vi "FlexMag - 23-03-2023.vi"() -> ()   [LabVIEW 2018] (continued)
  in  "Tp3 auto set speed":bool
  in  "Tp3 auto stop":bool
  in  "Tp3 auto start":bool
  in  "Tp4 auto normal speed":bool
  in  "Tp4 auto low speed":bool
  in  "Tp4 auto set speed":bool
  in  "Tp4 auto stop":bool
  in  "Tp4 auto start":bool
  in  "Tp1 Stop initial":bool
  in  "Tp1 Start initial":bool
  in  "Tp2 stop initial":bool
  in  "Tp2 start initial":bool
  in  "Tp3 stop initial":bool
  in  "Tp3 start initial":bool
  in  "Tp4 stop initial":bool
  in  "Tp4 start initial":bool
  out "Tp1_stop_cmnd":bool
  out "Tp2_stop_cmnd":bool
  out "Tp3_stop_cmnd":bool
  out "Tp4_stop_cmnd":bool
  out "tp1 com":bool
  out "tp2 com":bool
  out "tp3 com":bool
  out "tp4 com":bool
  in  "Adress set":bool
  out "after substring":string
  out "after substring 2":string
  out "after substring 3":string
  out "after substring 4":string
  out "tp3 readout":string
  out "tp2 readout":string
  out "tp1 readout":string
  out "tp4 readout":string
  in  "Baratron1 auto set zero":bool
  in  "pcgv1 auto set pressure":bool
  in  "pcgv1 auto close":bool
  in  "pcgv1 auto open":bool
  in  "pcgv1 auto set position":bool
  in  "Baratron2 auto set zero":bool
  in  "pcgv2 auto set pressure":bool
  in  "pcgv2 auto close":bool
  in  "pcgv2 auto set position":bool
  in  "pcgv2 auto open":bool
  in  "pcgv3 auto close":bool
  in  "pcgv3 auto set pressure":bool
  in  "pcgv3 auto set position":bool
  in  "Baratron3 set zero gui":bool
  in  "pcgv3 auto open":bool
  in  "Baratron4 auto set zero":bool
  in  "pcgv4 auto set pressure":bool
  in  "pcgv4 auto set position":bool
  in  "pcgv4 auto close":bool
  in  "pcgv4 auto open":bool
  out "pcgv1 setted pressure value torr":dbl
  out "pcgv2 setted pressure value torr":dbl
  out "pcgv3 setted pressure value torr":dbl
  out "pcgv4 setted pressure value torr":dbl
  in  "pcgv1 close gui 2":bool
  in  "pcgv1 open gui 2":bool
  in  "pcgv2 close gui 2":bool
  in  "pcgv2 open gui 2":bool
  in  "pcgv3 close gui 2":bool
  in  "pcgv3 open gui 2":bool
  in  "pcgv4 open gui 2":bool
  in  "pcgv4 close gui 2":bool
  in  "string":string
  in  "Learn":bool
  in  "Learn value":string
  out "Pressure_gui 2":dbl format="%.1f"
  out "Pressure_gui":dbl format="%.1f"
  out "Pressure":dbl format="%.1f"
  out "Pressure 2_gui 2":i32 format="%.1f"
  out "Pressure 2_gui":i32 format="%.1f"
  out "Pressure 2":i32 format="%.1f"
  out "Pressure ch3_gui2":i32 format="%.1f"
  out "Pressure ch3_gui":i32 format="%.1f"
  out "Pressure_ch3":i32
  out "Pressurech4_gui 2":i32 format="%.1f"
  out "Pressurech4_gui":i32 format="%.1f"
  out "Pressure 4":i32
  in  "Counter Data set":i16
  in  "Counter data set":bool
  out "Counter Read Data":i16
  out "CH1 CH BG":string
  out "CH2 CH BG":string
  out "CH4 CH BG":string
  out "CH3 CH BG":string
  out "CH1 CH CC":string
  out "CH1 CH PG":string
  out "ch4 pl pg torr":dbl format="%#_2e"
  out "ch4 pl pg mbar":dbl format="%#_2e"
  out "ch4 ch pg mbar":dbl format="%#_2e"
  out "ch4 ch pg torr":dbl format="%#_2e"
  out "ch4 cc torr":dbl format="%#_2e"
  out "ch4 cc mbar":dbl format="%#_2e"
  out "ch3 cc torr":dbl format="%#_2e"
  out "ch3 cc mbar":dbl format="%#_2e"
  out "ch3 ch pg torr":dbl format="%#_2e"
  out "ch3 ch pg mbar":dbl format="%#_2e"
  out "ch3 pl pg  torr":dbl format="%#_2e"
  out "ch3 pl pg mbar":dbl format="%#_2e"
  out "ch2 pl pg  torr":dbl format="%#_2e"
  out "ch2 pl pg mbar":dbl format="%#_2e"
  out "ch2 ch pg mbar":dbl format="%#_2e"
  out "ch2 ch pg torr":dbl format="%#_2e"
  out "ch2 cc torr":dbl format="%#_2e"
  out "ch2 cc mbar":dbl format="%#_2e"
  out "ch1 pl pg  torr":dbl format="%#_2e"
  out "ch1 pl pg mbar":dbl format="%#_2e"
  out "ch1 ch pg torr":dbl format="%#_2e"
  out "ch1 ch pg mbar":dbl format="%#_2e"
  out "ch1 cc torr":dbl format="%#_2e"
  out "ch1 cc mbar":dbl format="%#_2e"
  out "ch4 pl pg mbar gui 1":dbl format="%#_2e"
  out "ch3 pl pg mbar gui 1":dbl format="%#_2e"
  out "ch2 pl pg mbar gui 1":dbl format="%#_2e"
  out "ch1 pl pg mbar gui 1":dbl format="%#_2e"
  out "ch3 pl pg ai(V)":dbl
  out "ch3 ch pg ai(V)":dbl
  out "ch3 cc ai(V)":dbl
  out "ch2 pl pg ai(V)":dbl
  out "ch2 ch pg ai(V)":dbl
  out "ch2 cc ai(V)":dbl
  out "ch1 cc ai(V)":dbl
  out "ch1 ch pg ai(V)":dbl
  out "ch1 pl pg ai(V)":dbl
  out "ch4 pl pg ai(V)":dbl
  out "ch4 ch pg ai(V)":dbl
  out "ch4 cc ai(V)":dbl
  out "iteration for graph":i32
  out "hour s":string
  out "min s":string
  out "sec s":string
  out "hour":i32
  out "min":i32
  out "sec":i32
  out "time string":string
  out "CH1 PL PG":string
  out "CH2 CH CC":string
  out "CH2 CH PG":string
  out "CH2 PL PG":string
  out "CH4 CH CC":string
  out "CH4 CH PG":string
  out "CH4 PL PG":string
  out "CH3 CH CC":string
  out "CH3 CH PG":string
  out "CH3 PL PG":string
  in  "time  (sec)":u32
  in  "ch4 sd clear":bool
  in  "ch3 sd clear":bool
  in  "ch2 sd clear":bool
  in  "ch1 sd clear":bool
  in  "ch4 pd clear":bool
  in  "ch3 pd clear":bool
  in  "ch2 pd clear":bool
  in  "ch1 pd clear":bool
  out "ch1 pd continue":bool
  out "ch1 pd cancel":bool
  out "ch2 pd cancel":bool
  out "ch2 pd continue":bool
  out "ch3 pd cancel":bool
  out "ch3 pd continue":bool
  out "ch4 pd cancel":bool
  out "ch4 pd continue":bool
  out "ch1 sd cancel":bool
  out "ch1 sd continue":bool
  in  "ch1 shutdown alg":bool
  in  "ch2 shutdown alg":bool
  in  "ch4 shutdown alg":bool
  in  "ch3 shutdown alg":bool
  out "ch2 sd cancel":bool
  out "ch2 sd continue":bool
  out "ch3 sd cancel":bool
  out "ch3 sd continue":bool
  out "ch4 sd cancel":bool
  out "ch4 sd continue":bool
  in  "abort ch1":bool
  in  "abort ch2":bool
  in  "abort ch4":bool
  in  "abort ch3":bool
  in  "ch1 pumpdown alg":bool
  in  "ch2 pumpdown alg":bool
  in  "ch4 pumpdown alg":bool
  in  "ch3 pumpdown alg":bool
  in  "ch1 pumpdown error":bool
  in  "ch2 pumpdown error":bool
  in  "ch4 pumpdown error":bool
  in  "ch3 pumpdown error":bool
  in  "ch4 shutdown error":bool
  in  "ch3 shutdown error":bool
  in  "ch2 shutdown error":bool
  in  "ch1 shutdown error":bool
  out "ch1 vent?":bool
  out "ch2 vent?":bool
  out "ch3 vent?":bool
  out "ch4 vent?":bool
  out "ch1 atms close led":bool
  out "ch1 ch vbv close led":bool
  out "ch1 tp bv open led":bool
  out "ch1 pl vbv close led":bool
  out "ch1-ch2 trns gv close led 2":bool
  out "ch1 trns bp left close led":bool
  out "ch1 mp start led":bool
  out "ch1 pc gv open led":bool
  out "ch1 pl press under 0.05 T led":bool
  out "ch1 ch press under 0.5 T led":bool
  out "ch1 tp start led":bool
  out "ch1 trns bp left open led":bool
  out "ch1 ch press under 0.01 T led":bool
  out "ch1 cc open led":bool
  out "ch1 desired pressure led":bool
  out "ch1 pd completed led":bool
  out "ch1 sd completed led":bool
  out "ch1 sd PL-CH atm on led":bool
  out "ch1 sd PL atm on led":bool
  out "ch1 sd trns bp left close led":bool
  out "ch1 sd ch vbv open led":bool
  out "ch1 sd trns bp left open led":bool
  out "ch1 sd pcgv close led":bool
  out "ch1 sd atms close led":bool
  out "ch1 sd tp bv close led":bool
  out "ch1 sd pcgv open led":bool
  out "ch1 sd pl vbv open led":bool
  out "ch1 sd mp stop led":bool
  out "ch1 sd bg bv close led":bool
  out "ch1 sd tp stop led":bool
  out "ch1 sd cc close led":bool
  out "ch2 desired pressure led":bool
  out "ch2 cc open led":bool
  out "ch2 ch press under 0.01 T led":bool
  out "ch2 trns bp left open led":bool
  out "ch2 tp start led":bool
  out "ch2 ch press under 0.5 T led":bool
  out "ch2 pl press under 0.05 T led":bool
  out "ch1-ch2 trns gv close led":bool
  out "ch2 trns bp left close led":bool
  out "ch2 mp start led":bool
  out "ch2 pc gv open led":bool
  out "ch2 tp bv open led":bool
  out "ch2 pl vbv close led":bool
  out "ch2 ch vbv close led":bool
  out "ch2 atms close led":bool
  out "ch2 pd completed led":bool
  out "ch2 trns bp right close led":bool
  out "ch2 trns bp right open led":bool
  out "ch2-ch3 trns gv close led":bool
  out "ch2 sd completed led":bool
  out "ch2 sd PL-CH atm on led":bool
  out "ch2 sd PL atm on led":bool
  out "ch2 sd trns bp left close led":bool
  out "ch2 sd ch vbv open led":bool
  out "ch2 sd trns bp left open led":bool
  out "ch2 sd pcgv close led":bool
  out "ch2 sd atms close led":bool
  out "ch2 sd tp bv close led":bool
  out "ch2 sd pcgv open led":bool
  out "ch2 sd pl vbv open led":bool
  out "ch2 sd mp stop led":bool
  out "ch2 sd bg bv close led":bool
  out "ch2 sd tp stop led":bool
  out "ch2 sd cc close led":bool
  out "ch2 sd trns bp right close led":bool
  out "ch2 sd trns bp right open led":bool
  out "ch3 trns bp right open led":bool
  out "ch3 trns bp right close led":bool
  out "ch3 pd completed led":bool
  out "ch3 desired pressure led":bool
  out "ch3 cc open led":bool
  out "ch3 ch press under 0.01 T led":bool
  out "ch3 trns bp left open led":bool
  out "ch3 tp start led":bool
  out "ch3 ch press under 0.5 T led":bool
  out "ch3 pl press under 0.05 T led":bool
  out "ch3-ch2 trns gv close led":bool
  out "ch3 trns bp left close led":bool
  out "ch3 mp start led":bool
  out "ch3 pc gv open led":bool
  out "ch3 tp bv open led":bool
  out "ch3 pl vbv close led":bool
  out "ch3 ch vbv close led":bool
  out "ch3 atms close led":bool
  out "ch3-ch4 trns gv close led":bool
  out "ch4-ch3 trns gv close led":bool
  out "ch4 trns bp right open led":bool
  out "ch4 trns bp right close led":bool
  out "ch4 pd completed led":bool
  out "ch4 desired pressure led":bool
  out "ch4 cc open led":bool
  out "ch4 ch press under 0.01 T led":bool
  out "ch4 tp start led":bool
  out "ch4 ch press under 0.5 T led":bool
  out "ch4 pl press under 0.05 T led":bool
  out "ch4 mp start led":bool
  out "ch4 pc gv open led":bool
  out "ch4 tp bv open led":bool
  out "ch4 pl vbv close led":bool
  out "ch4 ch vbv close led":bool
  out "ch4 atms close led":bool
  out "ch3 sd trns bp right close led":bool
  out "ch3 sd trns bp right open led":bool
  out "ch3 sd completed led":bool
  out "ch3 sd PL-CH atm on led":bool
  out "ch3 sd PL atm on led":bool
  out "ch3 sd trns bp left close led":bool
  out "ch3 sd ch vbv open led":bool
  out "ch3 sd trns bp left open led":bool
  out "ch3 sd pcgv close led":bool
  out "ch3 sd atms close led":bool
  out "ch3 sd tp bv close led":bool
  out "ch3 sd pcgv open led":bool
  out "ch3 sd pl vbv open led":bool
  out "ch3 sd mp stop led":bool
  out "ch3 sd bg bv close led":bool
  out "ch3 sd tp stop led":bool
  out "ch3 sd cc close led":bool
  out "ch4 sd completed led":bool
  out "ch4 sd PL-CH atm on led":bool
  out "ch4 sd PL atm on led":bool
  out "ch4 sd trns bp right close led":bool
  out "ch4 sd ch vbv open led":bool
  out "ch4 sd trns bp right open led":bool
  out "ch4 sd pcgv close led":bool
  out "ch4 sd atms close led":bool
  out "ch4 sd tp bv close led":bool
  out "ch4 sd pcgv open led":bool
  out "ch4 sd pl vbv open led":bool
  out "ch4 sd mp stop led":bool
  out "ch4 sd bg bv close led":bool
  out "ch4 sd tp stop led":bool
  out "ch4 sd cc close led":bool
  in  "ch1 ar set zero auto":bool
  in  "ch1 ar set auto":bool
  in  "ch3 ar set auto":bool
  in  "ch2 ar set auto":bool
  in  "ch3 ar set zero auto":bool
  in  "ch2 ar set zero auto":bool
  in  "ch4 ar set zero auto":bool
  in  "ch4 ar set auto":bool
  in  "dewar error time(min)":dbl=10.0
  in  "error level":dbl=30.0
  in  "ln2 ch4 bottom drop":dbl=35.0
  in  "ln2 ch4 top aim":dbl=39.0
  in  "ln2 ch3 bottom drop":dbl=35.0
  in  "ln2 ch3 top aim":dbl=39.0
  in  "ln2 ch1 bottom drop":dbl=35.0
  in  "ln2 ch1 top aim":dbl=39.0
  in  "ln2 ch2 bottom drop":dbl=35.0
  in  "ln2 ch2 top aim":dbl=39.0
  in  "ln2 dropdown":dbl=32.0
  in  "GUI_inputs":enum32{"CH1", "CH2", "CH3", "CH4", "Others"}(tab)
  in  "ch1_mp_gui":bool
  in  "ch1_mp_fail":bool
  in  "ch1_pl_vbv_fail":bool
  in  "ch1_pl_vbv_gui":bool
  in  "ch1_pl_atm_fail":bool
  in  "ch1_pl_atm_gui":bool
  in  "ch1_pl_pg_fail":bool
  in  "ch1_pl_pg_gui":bool
  in  "ch1_tp_bv_fail":bool
  in  "ch1_tp_bv_gui":bool
  in  "ch1_ch_vbv_fail":bool
  in  "ch1_ch_vbv_gui":bool
  in  "ch1_tp_fail":bool
  in  "ch1_tp_gui":bool
  in  "ch1_pcgv_gui":bool
  in  "ch1_pcgv_half_gui":bool
  in  "ch1_pcgv_fail":bool
  in  "ch1_ch_pg_fail":bool
  in  "ch1_ch_pg_gui":bool
  in  "ch1_cc_fail":bool
  in  "ch1_cc_gui":bool
  in  "ch1_bg_fail":bool
  in  "ch1_bg_gui":bool
  in  "ch1_bg_bv_fail":bool
  in  "ch1_bg_bv_gui":bool
  in  "ch1_ch_atm_fail":bool
  in  "ch1_ch_atm_gui":bool
  in  "ch1_sov_fail":bool
  in  "ch1_sov_gui":bool
  in  "ch2_mp_fail":bool
  in  "ch2_mp_gui":bool
  in  "ch2_pl_vbv_fail":bool
  in  "ch2_pl_vbv_gui":bool
  in  "ch2_pl_atm_fail":bool
  in  "ch2_pl_atm_gui":bool
  in  "ch2_pl_pg_fail":bool
  in  "ch2_pl_pg_gui":bool
  in  "ch2_tp_bv_fail":bool
  in  "ch2_tp_bv_gui":bool
  in  "ch2_ch_vbv_fail":bool
  in  "ch2_ch_vbv_gui":bool
  in  "ch2_tp_fail":bool
  in  "ch2_tp_gui":bool
  in  "ch2_pcgv_gui":bool
  in  "ch2_pcgv_half_gui":bool
  in  "ch2_pcgv_fail":bool
  in  "ch2_ch_pg_fail":bool
  in  "ch2_ch_pg_gui":bool
  in  "ch2_cc_fail":bool
  in  "ch2_cc_gui":bool
  in  "ch2_bg_fail":bool
  in  "ch2_bg_gui":bool
  in  "ch2_bg_bv_fail":bool
  in  "ch2_bg_bv_gui":bool
  in  "ch2_ch_atm_fail":bool
  in  "ch2_ch_atm_gui":bool
  in  "ch2_sov_fail":bool
  in  "ch2_sov_gui":bool
  in  "ch3_mp_fail":bool
  in  "ch3_mp_gui":bool
  in  "ch3_pl_vbv_fail":bool
  in  "ch3_pl_vbv_gui":bool
  in  "ch3_pl_atm_fail":bool
  in  "ch3_pl_atm_gui":bool
  in  "ch3_pl_pg_fail":bool
  in  "ch3_pl_pg_gui":bool
  in  "ch3_tp_bv_fail":bool
  in  "ch3_tp_bv_gui":bool
  in  "ch3_ch_vbv_fail":bool
  in  "ch3_ch_vbv_gui":bool
  in  "ch3_tp_fail":bool
  in  "ch3_tp_gui":bool
  in  "ch3_pcgv_half_gui":bool
  in  "ch3_pcgv_gui":bool
  in  "ch3_pcgv_fail":bool
  in  "ch3_ch_pg_fail":bool
  in  "ch3_ch_pg_gui":bool
  in  "ch3_cc_fail":bool
  in  "ch3_cc_gui":bool
  in  "ch3_bg_fail":bool
  in  "ch3_bg_gui":bool
  in  "ch3_bg_bv_fail":bool
  in  "ch3_bg_bv_gui":bool
  in  "ch3_ch_atm_fail":bool
  in  "ch3_ch_atm_gui":bool
  in  "ch3_sov_fail":bool
  in  "ch3_sov_gui":bool
  in  "ch4_mp_fail":bool
  in  "ch4_mp_gui":bool
  in  "ch4_pl_vbv_fail":bool
  in  "ch4_pl_vbv_gui":bool
  in  "ch4_pl_atm_fail":bool
  in  "ch4_pl_atm_gui":bool
  in  "ch4_pl_pg_fail":bool
  in  "ch4_pl_pg_gui":bool
  in  "ch4_tp_bv_fail":bool
  in  "ch4_tp_bv_gui":bool
  in  "ch4_ch_vbv_fail":bool
  in  "ch4_ch_vbv_gui":bool
  in  "ch4_tp_fail":bool
  in  "ch4_tp_gui":bool
  in  "ch4_pcgv_gui":bool
  in  "ch4_pcgv_half_gui":bool
  in  "ch4_pcgv_fail":bool
  in  "ch4_ch_pg_fail":bool
  in  "ch4_ch_pg_gui":bool
  in  "ch4_cc_fail":bool
  in  "ch4_cc_gui":bool
  in  "ch4_bg_fail":bool
  in  "ch4_bg_gui":bool
  in  "ch4_bg_bv_fail":bool
  in  "ch4_bg_bv_gui":bool
  in  "ch4_ch_atm_fail":bool
  in  "ch4_ch_atm_gui":bool
  in  "ch4_sov_fail":bool
  in  "ch4_sov_gui":bool
  in  "ch3_4_trns_gv_fail":bool
  in  "ch3_4_trns_gv_gui":bool
  in  "ch2_3_trns_gv_fail":bool
  in  "ch2_3_trns_gv_gui":bool
  in  "ch1_2_trns_gv_fail":bool
  in  "ch1_2_trns_gv_gui":bool
  in  "ch4_gv_bp_right_fail":bool
  in  "ch4_gv_bp_right_gui":bool
  in  "ch3_gv_bp_right_fail":bool
  in  "ch3_gv_bp_right_gui":bool
  in  "ch2_gv_bp_right_fail":bool
  in  "ch2_gv_bp_right_gui":bool
  in  "ch3_gv_bp_left_fail":bool
  in  "ch3_gv_bp_left_gui":bool
  in  "ch2_gv_bp_left_fail":bool
  in  "ch2_gv_bp_left_gui":bool
  in  "ch1_gv_bp_left_fail":bool
  in  "ch1_gv_bp_left_gui":bool
  in  "casette_ch1_gui":bool
  in  "casette_ch3_gui":bool
  in  "casette_ch2_gui":bool
  in  "casette_ch4_gui":bool
  in  "24-bit pixmap tab":enum32{"Page 1", "Page 2", "Page 3", "Page 4"}(tab)
  out "main screen jpeg":u32[][](array[numeric]) format="%x"
  out "pl pg fail jpeg":u32[][](array[numeric]) format="%x"
  out "pl pg on jpeg":u32[][](array[numeric]) format="%x"
  out "pc gv half jpeg":u32[][](array[numeric]) format="%x"
  out "cc fail jpeg":u32[][](array[numeric]) format="%x"
  out "cc on jpeg":u32[][](array[numeric]) format="%x"
  out "gv bp left fail jpeg":u32[][](array[numeric]) format="%x"
  out "gv bp left on jpeg":u32[][](array[numeric]) format="%x"
  out "tp bv fail jpeg":u32[][](array[numeric]) format="%x"
  out "tp bv on jpeg":u32[][](array[numeric]) format="%x"
  out "pc gv fail jpeg":u32[][](array[numeric]) format="%x"
  out "pc gv on jpeg":u32[][](array[numeric]) format="%x"
  out "bg fail jpeg":u32[][](array[numeric]) format="%x"
  out "bg on jpeg":u32[][](array[numeric]) format="%x"
  out "gv bp right fail jpeg":u32[][](array[numeric]) format="%x"
  out "gv bp right on jpeg":u32[][](array[numeric]) format="%x"
  out "ch pg on jpeg":u32[][](array[numeric]) format="%x"
  out "ch pg fail jpeg":u32[][](array[numeric]) format="%x"
  out "pl atm on jpeg":u32[][](array[numeric]) format="%x"
  out "pl atm fail jpeg":u32[][](array[numeric]) format="%x"
  out "ch atm on jpeg":u32[][](array[numeric]) format="%x"
  out "ch atm fail jpeg":u32[][](array[numeric]) format="%x"
  out "tp start jpeg":u32[][](array[numeric]) format="%x"
  out "tp fail jpeg":u32[][](array[numeric]) format="%x"
  out "pl vbv fail jpeg":u32[][](array[numeric]) format="%x"
  out "pl vbv on jpeg":u32[][](array[numeric]) format="%x"
  out "bg bv on jpeg":u32[][](array[numeric]) format="%x"
  out "bg bv fail jpeg":u32[][](array[numeric]) format="%x"
  out "tp vbv on jpeg":u32[][](array[numeric]) format="%x"
  out "tp vbv fail jpeg":u32[][](array[numeric]) format="%x"
  out "mp on jpeg":u32[][](array[numeric]) format="%x"
  out "mp fail jpeg":u32[][](array[numeric]) format="%x"
  out "trns gv fail jpeg":u32[][](array[numeric]) format="%x"
  out "trns gv on jpeg":u32[][](array[numeric]) format="%x"
  out "ch1 top main jpeg":u32[][](array[numeric]) format="%x"
  out "ch1 front main jpeg":u32[][](array[numeric]) format="%x"
  out "ch2 front main jpeg":u32[][](array[numeric]) format="%x"
  out "ch2 top main jpeg":u32[][](array[numeric]) format="%x"
  out "ch3 front main jpeg":u32[][](array[numeric]) format="%x"
  out "ch3 top main jpeg":u32[][](array[numeric]) format="%x"
  out "ch4 front main jpeg":u32[][](array[numeric]) format="%x"
  out "ch4 top main jpeg":u32[][](array[numeric]) format="%x"
  out "sov fail jpeg":u32[][](array[numeric]) format="%x"
  out "sov on jpeg":u32[][](array[numeric]) format="%x"
  out "trns gv top right fail jpeg":u32[][](array[numeric]) format="%x"
  out "trns gv top right on  jpeg":u32[][](array[numeric]) format="%x"
  out "trns gv front left on jpeg":u32[][](array[numeric]) format="%x"
  out "trns gv front left fail jpeg":u32[][](array[numeric]) format="%x"
  out "trns gv front right on jpeg":u32[][](array[numeric]) format="%x"
  out "trns gv front right fail jpeg":u32[][](array[numeric]) format="%x"
  out "trns gv top left fail jpeg":u32[][](array[numeric]) format="%x"
  out "trns gv top left on jpeg":u32[][](array[numeric]) format="%x"
  out "casette jpeg":u32[][](array[numeric]) format="%x"
  out "trns sensors led":bool
  in  "deactivate all trns sensors":bool
  in  "Cst_Speed_Low":dbl=500.0
  out "trns V?":bool
  out "trns 2-3 led 1":bool
  out "trns 2-3 led 4":bool
  out "trns 2-3 led 6":bool
  out "trns 2-3 led 8":bool
  out "trns 2-3 led 2":bool
  out "trns 2-3 led 3":bool
  out "trns 2-3 led 5":bool
  out "trns 2-3 led 7":bool
  out "trns 2-3 led 9":bool
  out "trns 2-3 led 10":bool
  out "trns 2-3 led 11":bool
  out "trns 2-3 led 12":bool
  out "trns 2-3 led 13":bool
  out "trns 2-3 led 14":bool
  out "trns 2-3 led 15":bool
  out "trns 2-3 led 16":bool
  out "trns 2-3 led 17":bool
  out "trns 2-3 led 18":bool
  out "trns 2-3 led 19":bool
  out "trns 2-3 led 20":bool
  out "trns 2-3 led 22":bool
  out "trns 2-3 led 21":bool
  out "trns 2-3 led 23":bool
  out "trns 2-3 led 24":bool
  out "trns pre check led 1":bool
  in  "trns error":bool
  in  "trns pre check":bool
  in  "ch1-2 transfer":bool
  out "TRNS atm alg":bool
  in  "transfer vacuum auto":bool
  in  "transfer atm auto":bool
  out "TRNS vacuum alg":bool
  in  "ch2-3 transfer":bool
  in  "ch2-1 transfer":bool
  in  "ch3-2 transfer":bool
  in  "ch4-3 transfer":bool
  in  "ch3-4 transfer":bool
  out "1-2 tr":bool
  out "1-3 tr":bool
  out "1-4 tr":bool
  out "2-1 tr":bool
  out "2-3 tr":bool
  out "2-4 tr":bool
  out "3-1 tr":bool
  out "3-2 tr":bool
  out "3-4 tr":bool
  out "4-3 tr":bool
  out "4-1 tr":bool
  out "4-2 tr":bool
  out "trns pre check led 2":bool
  out "trns pre check led 3":bool
  out "trns pre check led 4":bool
  out "trns pre check led 5":bool
  out "trns pre check led 6":bool
  out "trns pre check led 7":bool
  out "trns pre check led 8":bool
  out "trns pre check led 9":bool
  out "trns pre check led 10":bool
  out "trns pre check led 11":bool
  out "trns pre check led 12":bool
  in  "trns clear":bool
  out "trns 1-2 led 1":bool
  out "trns 1-2 led 2":bool
  out "trns 1-2 led 3":bool
  out "trns 1-2 led 4":bool
  out "trns 1-2 led 7":bool
  out "trns 1-2 led 8":bool
  out "trns 1-2 led 6":bool
  out "trns 1-2 led 5":bool
  out "trns 1-2 led 9":bool
  out "trns 1-2 led 10":bool
  out "trns 1-2 led 11":bool
  out "trns 1-2 led 12":bool
  out "trns 1-2 led 13":bool
  out "trns 1-2 led 14":bool
  out "trns 1-2 led 15":bool
  out "trns 1-2 led 16":bool
  out "trns 1-2 led 17":bool
  out "trns 1-2 led 18":bool
  out "trns 1-2 led 19":bool
  out "trns 1-2 led 20":bool
  out "trns 1-2 led 21":bool
  out "trns 1-2 led 22":bool
  out "trns 1-2 led 23":bool
  out "trns 3-4 led 24":bool caption="trns 2-3 led 24"
  out "trns 3-4 led 23":bool caption="trns 2-3 led 23"
  out "trns 3-4 led 21":bool caption="trns 2-3 led 21"
  out "trns 3-4 led 22":bool caption="trns 2-3 led 22"
  out "trns 3-4 led 20":bool caption="trns 2-3 led 20"
  out "trns 3-4 led 19":bool caption="trns 2-3 led 19"
  out "trns 3-4 led 18":bool caption="trns 2-3 led 18"
  out "trns 3-4 led 17":bool caption="trns 2-3 led 17"
  out "trns 3-4 led 13":bool caption="trns 2-3 led 13"
  out "trns 3-4 led 14":bool caption="trns 2-3 led 14"
  out "trns 3-4 led 15":bool caption="trns 2-3 led 15"
  out "trns 3-4 led 16":bool caption="trns 2-3 led 16"
  out "trns 3-4 led 9":bool caption="trns 2-3 led 9"
  out "trns 3-4 led 10":bool caption="trns 2-3 led 10"
  out "trns 3-4 led 11":bool caption="trns 2-3 led 11"
  out "trns 3-4 led 12":bool caption="trns 2-3 led 12"
  out "trns 3-4 led 5":bool caption="trns 2-3 led 5"
  out "trns 3-4 led 6":bool caption="trns 2-3 led 6"
  out "trns 3-4 led 7":bool caption="trns 2-3 led 7"
  out "trns 3-4 led 8":bool caption="trns 2-3 led 8"
  out "trns 3-4 led 3":bool caption="trns 2-3 led 3"
  out "trns 3-4 led 4":bool caption="trns 2-3 led 4"
  out "trns 3-4 led 2":bool caption="trns 2-3 led 2"
  out "trns 3-4 led 1":bool caption="trns 2-3 led 1"
  out "trns 2-1 led 1":bool caption="trns 2-3 led 1"
  out "trns 2-1 led 2":bool caption="trns 2-3 led 2"
  out "trns 2-1 led 4":bool caption="trns 2-3 led 4"
  out "trns 2-1 led 3":bool caption="trns 2-3 led 3"
  out "trns 2-1 led 8":bool caption="trns 2-3 led 8"
  out "trns 2-1 led 7":bool caption="trns 2-3 led 7"
  out "trns 2-1 led 6":bool caption="trns 2-3 led 6"
  out "trns 2-1 led 5":bool caption="trns 2-3 led 5"
  out "trns 2-1 led 12":bool caption="trns 2-3 led 12"
  out "trns 2-1 led 11":bool caption="trns 2-3 led 11"
  out "trns 2-1 led 10":bool caption="trns 2-3 led 10"
  out "trns 2-1 led 9":bool caption="trns 2-3 led 9"
  out "trns 2-1 led 16":bool caption="trns 2-3 led 16"
  out "trns 2-1 led 15":bool caption="trns 2-3 led 15"
  out "trns 2-1 led 14":bool caption="trns 2-3 led 14"
  out "trns 2-1 led 13":bool caption="trns 2-3 led 13"
  out "trns 2-1 led 17":bool caption="trns 2-3 led 17"
  out "trns 2-1 led 18":bool caption="trns 2-3 led 18"
  out "trns 2-1 led 19":bool caption="trns 2-3 led 19"
  out "trns 2-1 led 20":bool caption="trns 2-3 led 20"
  out "trns 2-1 led 22":bool caption="trns 2-3 led 22"
  out "trns 2-1 led 21":bool caption="trns 2-3 led 21"
  out "trns 2-1 led 23":bool caption="trns 2-3 led 23"
  out "trns 2-1 led 24":bool caption="trns 2-3 led 24"
  out "trns 3-2 led 24":bool caption="trns 2-3 led 24"
  out "trns 3-2 led 23":bool caption="trns 2-3 led 23"
  out "trns 3-2 led 21":bool caption="trns 2-3 led 21"
  out "trns 3-2 led 22":bool caption="trns 2-3 led 22"
  out "trns 3-2 led 20":bool caption="trns 2-3 led 20"
  out "trns 3-2 led 19":bool caption="trns 2-3 led 19"
  out "trns 3-2 led 18":bool caption="trns 2-3 led 18"
  out "trns 3-2 led 17":bool caption="trns 2-3 led 17"
  out "trns 3-2 led 13":bool caption="trns 2-3 led 13"
  out "trns 3-2 led 14":bool caption="trns 2-3 led 14"
  out "trns 3-2 led 15":bool caption="trns 2-3 led 15"
  out "trns 3-2 led 16":bool caption="trns 2-3 led 16"
  out "trns 3-2 led 9":bool caption="trns 2-3 led 9"
  out "trns 3-2 led 10":bool caption="trns 2-3 led 10"
  out "trns 3-2 led 11":bool caption="trns 2-3 led 11"
  out "trns 3-2 led 12":bool caption="trns 2-3 led 12"
  out "trns 3-2 led 5":bool caption="trns 2-3 led 5"
  out "trns 3-2 led 6":bool caption="trns 2-3 led 6"
  out "trns 3-2 led 7":bool caption="trns 2-3 led 7"
  out "trns 3-2 led 8":bool caption="trns 2-3 led 8"
  out "trns 3-2 led 3":bool caption="trns 2-3 led 3"
  out "trns 3-2 led 4":bool caption="trns 2-3 led 4"
  out "trns 3-2 led 2":bool caption="trns 2-3 led 2"
  out "trns 3-2 led 1":bool caption="trns 2-3 led 1"
  out "trns 4-3 led 23":bool caption="trns 2-3 led 23"
  out "trns 4-3 led 21":bool caption="trns 2-3 led 21"
  out "trns 4-3 led 22":bool caption="trns 2-3 led 22"
  out "trns 4-3 led 20":bool caption="trns 2-3 led 20"
  out "trns 4-3 led 19":bool caption="trns 2-3 led 19"
  out "trns 4-3 led 18":bool caption="trns 2-3 led 18"
  out "trns 4-3 led 17":bool caption="trns 2-3 led 17"
  out "trns 4-3 led 13":bool caption="trns 2-3 led 13"
  out "trns 4-3 led 14":bool caption="trns 2-3 led 14"
  out "trns 4-3 led 15":bool caption="trns 2-3 led 15"
  out "trns 4-3 led 16":bool caption="trns 2-3 led 16"
  out "trns 4-3 led 9":bool caption="trns 2-3 led 9"
  out "trns 4-3 led 10":bool caption="trns 2-3 led 10"
  out "trns 4-3 led 11":bool caption="trns 2-3 led 11"
  out "trns 4-3 led 12":bool caption="trns 2-3 led 12"
  out "trns 4-3 led 5":bool caption="trns 2-3 led 5"
  out "trns 4-3 led 6":bool caption="trns 2-3 led 6"
  out "trns 4-3 led 7":bool caption="trns 2-3 led 7"
  out "trns 4-3 led 8":bool caption="trns 2-3 led 8"
  out "trns 4-3 led 3":bool caption="trns 2-3 led 3"
  out "trns 4-3 led 4":bool caption="trns 2-3 led 4"
  out "trns 4-3 led 2":bool caption="trns 2-3 led 2"
  out "trns 4-3 led 1":bool caption="trns 2-3 led 1"
  in  "Cst_Speed_High":dbl=700.0
  in  "activate all trns sensors":bool
  in  "check both tensions":bool
  in  "speed compare value":sgl
  in  "speed check (sec)":sgl=15.0
  in  "speed check active":bool
  in  "tension check (sec)":sgl=7.0
  in  "tension check active":bool
  in  "rollback -1 ?":bool
  in  "cycle step count":sgl=10.0
  out "TC2_diameter_readout":sgl format="%#.3f"
  out "TC1_diameter_readout":sgl format="%#.3f"
  in  "roll error":bool
  in  "TC TAB":T7(tab)
  in  "TC1_reg_set":bool
  in  "TC1_setpoint_type":bool
  in  "TC1_regulation_type_value":sgl
  in  "TC1_regulation_type_selection":bool
  in  "TC1_tare_function":bool
  in  "TC1_display_tension_set":bool
  in  "TC1_display_AO1_set":bool
  in  "TC1_display_tension_actual":bool
  in  "TC1_display_AO1_actual":bool
  in  "TC1_set_value":sgl=10.0
  in  "TC1_set":bool
  in  "TC1_auto_set":bool
  out "TC2_Tension_read_set":u16
  out "TC1_Tension_read_set":u16
  out "TC1_readout_set_value":sgl format="%#.1f"
  out "TC1_measure_value":sgl format="%#.1f"
  in  "TC1_AO1_bottom_limit_value":sgl
  in  "TC1_AO1_upper_limit_value":sgl=10.0
  in  "TC1_overspeed_value":sgl=1.0
  in  "TC1_speed_coefficient_value":sgl=10.0
  in  "TC1_speed_gain_value":sgl=28.0
  in  "TC1_D_coefficient":sgl
  in  "TC1_I_coefficient":sgl=20.0
  in  "TC1_P_coefficient":sgl=100.0
  in  "TC1_close_loop_coefficient":sgl=100.0
  in  "TC1_open_loop_coefficient":sgl
  in  "TC1_open_loop_set":bool
  in  "TC1_close_loop_set":bool
  in  "TC1_P_set":bool
  in  "TC1_I_set":bool
  in  "TC1_D_set":bool
  in  "TC1_speed_gain_set":bool
  in  "TC1_speed_coefficient_set":bool
  in  "TC1_overspeed_set":bool
  in  "TC1_AO1_upper_limit_set":bool
  in  "TC1_AO1_bottom_limit_set":bool
  in  "TC1_AO1_polarity(neg_to_pos)":bool
  in  "TC1_AO1_polarity(pos_to_neg)":bool
  in  "TC1_setpoint_type_value":sgl
  in  "tc1 data set to reg":sgl
  in  "tc1 Starting Address":u16
  in  "TC2_setpoint_type_value":sgl
  in  "TC2_setpoint_type":bool
  in  "TC2_display_tension_set":bool
  in  "TC2_display_AO1_set":bool
  in  "TC2_tare_function":bool
  in  "TC2_display_tension_actual":bool
  in  "TC2_display_AO1_actual":bool
  in  "TC2_auto_set":bool
  in  "TC2_AO1_bottom_limit_value":sgl
  in  "TC2_AO1_upper_limit_value":sgl=10.0
  in  "TC2_overspeed_value":sgl=1.0
  in  "TC2_speed_coefficient_value":sgl=10.0
  in  "TC2_speed_gain_value":sgl=28.0
  in  "TC2_D_coefficient":sgl
  in  "TC2_I_coefficient":sgl=20.0
  in  "TC2_P_coefficient":sgl=100.0
  in  "TC2_close_loop_coefficient":sgl=100.0
  in  "TC2_open_loop_coefficient":sgl
  in  "TC2_set_value":sgl=10.0
  out "TC2_reading_set_value":sgl format="%#.1f"
  out "TC2_measure_value":sgl format="%#.1f"
  in  "TC2_open_loop_set":bool
  in  "TC2_close_loop_set":bool
  in  "TC2_P_set":bool
  in  "TC2_I_set":bool
  in  "TC2_D_set":bool
  in  "TC2_speed_gain_set":bool
  in  "TC2_speed_coefficient_set":bool
  in  "TC2_overspeed_set":bool
  in  "TC2_AO1_upper_limit_set":bool
  in  "TC2_AO1_bottom_limit_set":bool
  in  "TC2_AO1_polarity(neg_to_pos)":bool
  in  "TC2_AO1_polarity(pos_to_neg)":bool
  in  "TC2_regulation_type_value":sgl
  in  "TC2_regulation_type_selection":bool
  in  "TC2_set":bool
  in  "TC2_reg_set":bool
  in  "tc2 data set to reg":sgl
  in  "tc2 Starting Address":u16
  in  "pid output":bool
  in  "final output voltage":dbl
  in  "PID gains":T8={"proportional gain (Kc)"=0.0002, "integral time (Ti, min)"=0.0015, "derivative time (Td, min)"=0.0} {"derivative time (Td, min)" format="%.7f"; "integral time (Ti, min)" format="%.7f"; "proportional gain (Kc)" format="%.7f"}
  in  "dt (s)":dbl=-1.0 format="%.3f"
  in  "output range":cluster{"output high":dbl, "output low":dbl}={"output high"=10.0, "output low"=5.0} {"output low" format="%.2f"; "output high" format="%.2f"}
  out "output_pid":dbl format="%.6f"
  in  "decreasing voltage":dbl format="%#.5g"
  in  "initial output voltage":dbl
  out "min circular speed":dbl
  out "max circular speed":dbl
  in  "lap number right target":dbl
  in  "total interval":dbl
  in  "final right diameter":dbl
  in  "current voltage":dbl
  in  "show graph":bool
  in  "freq coef":sgl=182.0
  in  "speed coef":sgl=550.0
  in  "target interval":dbl=100.0
  in  "web speed":dbl=400.0
  in  "web thickness":dbl=50.0
  in  "initial right diameter":dbl=93.0
  in  "calculate":bool
  in  "lap number left target":dbl
  out "freq readout":dbl
  in  "TC parameter set":bool
  in  "Roll Forw":bool
  in  "waiting_TC":u32=500
  out "TC1_speed readout":sgl format="%#.3f"
  out "TC2_speed readout":sgl format="%#.3f"
  out "TC2_line speed readout":sgl format="%#.3f"
  out "TC1_line speed readout":sgl format="%#.3f"
  in  "tension check value":sgl=15.0
  in  "position":bool
  in  "set speed (ms)":u32=1000
  out "error out":errorcluster
  out "process counter":dbl
  in  "dep. for?":bool
  in  "coating clear":bool
  in  "Auto Deposition Leds":T9(tab)
  out "coating ch2 led 1":bool
  out "coating ch2 led 2":bool
  out "coating ch2 led 3":bool
  out "coating ch2 led 4":bool
  out "coating ch2 led 6":bool
  out "coating ch2 led 8":bool
  out "coating ch2 led 9":bool
  out "coating ch2 led 5":bool
  out "coating ch2 led 10":bool
  out "coating ch2 led 7":bool
  out "coating ch2 led 11":bool
  out "coating ch2 led 12":bool
  out "coating ch2 led 13":bool
  out "coating ch2 led 14":bool
  out "coating ch2 led 15":bool
  out "coating ch2 led 16":bool
  out "coating ch2 led 17":bool
  out "coating ch2 led 18":bool
  out "coating ch2 led 19":bool
  out "coating ch2 led 20":bool
  out "coating ch3 led 1":bool
  out "coating ch3 led 2":bool
  out "coating ch3 led 3":bool
  out "coating ch3 led 4":bool
  out "coating ch3 led 5":bool
  out "coating ch3 led 6":bool
  out "coating ch3 led 7":bool
  out "coating ch3 led 8":bool
  out "coating ch3 led 9":bool
  out "coating ch3 led 10":bool
  out "coating ch3 led 11":bool
  out "coating ch3 led 12":bool
  out "coating ch3 led 13":bool
  out "coating ch3 led 14":bool
  out "coating ch3 led 15":bool
  out "coating ch3 led 16":bool
  out "coating ch3 led 17":bool
  out "coating ch3 led 18":bool
  out "coating ch3 led 19":bool
  out "coating ch3 led 20":bool
  out "coating ch4 led 1":bool
  out "coating ch4 led 2":bool
  out "coating ch4 led 3":bool
  out "coating ch4 led 4":bool
  out "coating ch4 led 5":bool
  out "coating ch4 led 6":bool
  out "coating ch4 led 7":bool
  out "coating ch4 led 8":bool
  out "coating ch4 led 9":bool
  out "coating ch4 led 10":bool
  out "coating ch4 led 11":bool
  out "coating ch4 led 12":bool
  out "coating ch4 led 13":bool
  out "coating ch4 led 14":bool
  out "coating ch4 led 15":bool
  out "coating ch4 led 16":bool
  out "coating ch4 led 17":bool
  out "coating ch4 led 18":bool
  out "coating ch4 led 19":bool
  out "coating ch4 led 20":bool
  out "time counting":dbl
  in  "coating error":bool
  in  "coating process done":bool
  in  "roll error (min)":i32=40
  out "forroll stop cmd":bool
  out "backroll stop cmd":bool
  in  "step count 2":dbl
  in  "write":bool
  in  "QR save":bool
  in  "QR reset":bool
  out "qr read buffer if available":string
  out "read buffer always":string
  in  "read":bool
  in  "QR off mode":bool
  in  "QR continuous mode":bool
  out "qr read statue":string
  out "read if asked":string
  in  "write buffer":string
  out "error out 2":errorcluster
  in  "qr wait second":u32=5
  in  "gui tab buttons":enum32{"CH1", "CH2", "CH3", "CH4"}(tab)
  in  "CH1-2 trns close gui 1":bool
  in  "CH1-2 trns open gui 1":bool
  in  "ch1 trnsbp left open gui1":bool
  in  "ch1 trnsbp left close gui 1":bool
  in  "Tp1 stop gui 1":bool
  in  "Tp1 start gui 1":bool
  in  "pcgv1 open gui 1":bool
  in  "pcgv1 close gui 1":bool
  in  "chvbv1 open gui 1":bool
  in  "chvbv1 close gui 1":bool
  in  "plvbv1 open gui 1":bool
  in  "plvbv1 close gui 1":bool
  in  "mp1 start gui 1":bool
  in  "mp1 stop gui 1":bool
  in  "tpbv1 open gui 1":bool
  in  "tpbv1 close gui 1":bool
  in  "bgbv1 open gui 3":bool
  in  "bgbv1 close gui 1":bool
  in  "cc1 open gui 1":bool
  in  "cc1 close gui 1":bool
  in  "CH1-2 trns close gui 2":bool
  in  "CH1-2 trns open gui 2":bool
  in  "pcgv2 open gui 1":bool
  in  "pcgv2 close gui 1":bool
  in  "chvbv2 close gui 1":bool
  in  "chvbv2 open gui 1":bool
  in  "plvbv2 close gui 1":bool
  in  "plvbv2 open gui 1":bool
  in  "mp2 stop gui 1":bool
  in  "mp2 start gui 1":bool
  in  "tpbv2 close gui 1":bool
  in  "tpbv2 open gui 1":bool
  in  "ch2 trnsbp left close gui 1":bool
  in  "ch2 trnsbp left open gui 1":bool
  in  "ch2 trnsbp right close gui 1":bool
  in  "ch2 trnsbp right open gui 1":bool
  in  "Tp2 start gui 1":bool
  in  "Tp2 stop gui 1":bool
  in  "cc2 close gui 1":bool
  in  "cc2 open gui 1":bool
  in  "bgbv2 close gui 1":bool
  in  "bgbv1 open gui 1":bool
  in  "CH2-3 trns close gui 1":bool
  in  "CH2-3 trns open gui 1":bool
  in  "CH3-4 trns close gui 1":bool
  in  "CH3-4 trns open gui 1":bool
  in  "CH2-3 trns open gui 2":bool
  in  "CH2-3 trns close gui 2":bool
  in  "ch3 trnsbp right open gui 1":bool
  in  "ch3 trnsbp right close gui 1":bool
  in  "Tp3 start gui 1":bool
  in  "Tp3 stop gui 1":bool
  in  "pcgv3 close gui 1":bool
  in  "pcgv3 open gui 1":bool
  in  "cc3 open gui 1":bool
  in  "cc3 close gui 1":bool
  in  "chvbv3 open gui 1":bool
  in  "chvbv3 close gui 1":bool
  in  "tpbv3 open gui 1":bool
  in  "tpbv3 close gui 1":bool
  in  "plvbv3 close gui 1":bool
  in  "plvbv3 open gui 1":bool
  in  "mp3 stop gui 1":bool
  in  "mp3 start gui 1":bool
  in  "bgbv3 open gui 1":bool
  in  "bgbv3 close gui 1":bool
  in  "ch3 trnsbp left open gui 1":bool
  in  "ch3 trnsbp left close gui 1":bool
  in  "CH3-4 trns close gui 2":bool
  in  "CH3-4 trns open gui 2":bool
  in  "ch4 trnsbp right close gui 1":bool
  in  "ch4 trnsbp right open gui 1":bool
  in  "Tp4 start gui 1":bool
  in  "Tp4 stop gui 1":bool
  in  "pcgv4 open gui 1":bool
  in  "pcgv4 close gui 1":bool
  in  "cc4 close gui 1":bool
  in  "cc4 open gui 1":bool
  in  "tpbv4 close gui 1":bool
  in  "tpbv4 open gui 1":bool
  in  "plvbv4 close gui 1":bool
  in  "plvbv4 open gui 1":bool
  in  "mp4 stop gui 1":bool
  in  "mp4 start gui 1":bool
  in  "chvbv4 close gui 1":bool
  in  "chvbv4 open gui 1":bool
  in  "bgbv4 close gui 1":bool
  in  "bgbv4 open gui 1":bool
  out "read from keysight CASE 1":string
  out "keysight readout 2":dbl
  in  "keysight case 1":string="*IDN?\n"
  in  "case1":bool
  in  "output limit min":dbl
  in  "output limit max":dbl=500.0
  out "error out keysight":errorcluster
  in  "keysight default case":string="MEAS:FREQ?\n"
  out "read from keysight":string
  in  "keysight loop (ms)":u32=300
  out "keysight readout":dbl
  in  "keysight wait time":u32=100
  # "DCPS MAG\nSELECTION"
  # "DESCRIPTION"
  # "SYSTEM STATUS"
  # "NONE"
  # "WARNING\nMESSAGES"
  # "web speed"
  # "core diameter"
  # "left initial diameter"
  # "tension"
  # "web thickness"
  # "DC Sputtering"
  # "RF Sputtering"
  # "Step Number"
  # "Power"
  # "Step Number"
  # "Length"
  # "Power"
  # "Length"
  # "Microwave Power"
  # "Hz"
  # "Hz"
  # "Hz"
  # "Hz"
  # "CH4"
  # "CH3"
  # "CH2"
  # "CH1"
  # "Cassette Position"
  # "Pressure Graph"
  # "sec"
  # "TRANSFER CONTROL"
  # "TARGET CHAMBER"
  # "PRESENT LOCATION"
  # "TURBO PUMP CONTROL"
  # "AUTOMATIC PROCESS"
  # "DESIRED\nPRESSURE"
  # "mbarr"
  # "TURBO PUMP CONTROL"
  # "AUTOMATIC PROCESS"
  # "DESIRED\nPRESSURE"
  # "mbarr"
  # "TURBO PUMP CONTROL"
  # "AUTOMATIC PROCESS"
  # "DESIRED\nPRESSURE"
  # "mbarr"
  # "AUTOMATIC PROCESS"
  # "DESIRED\nPRESSURE"
  # "mbarr"
  # "TURBO PUMP CONTROL"
  # "Q R      S C A N N E R"
  # "R O L L I N G     P A R A M E T E R S"
  # "Tension Value"
  # "N"
  # "Actual Speed"
  # "cm/min"
  # "Set Speed"
  # "cm/min"
  # "Current Step"
  # "Step Number"
  # "Lap Number R Actual"
  # "lap"
  # "Lap Number L Actual"
  # "Max  Lap Number"
  # "lap"
  # "P I S T O N S     P O S I T I O N"
  # "CST-FIX"
  # "PETCOOL"
  # "SRV-PISTON"
  # "CH1"
  # "CH2"
  # "CH3"
  # "CH4"
  # "R O L L I N G     C O N T R O L"
  # "TENSION\nCONTROLLER\nSTATUS"
  # "P I S T O N S     C O N T R O L"
  # "CH1"
  # "CH2"
  # "CH3"
  # "CH4"
  # "C Y C L E     R O L L"
  # "Number of Cycle"
  # "Remaining Cycle"
  # "Recipe & Process Files"
  # "Automatic Deposition"
  # "Rolling Direction"
  # "Controls"